vi "UHR-Fleezers Control (host) - 10.3.vi"() -> ()   [LabVIEW 2010]
uses:
  <vilib>/Utility/miscctls.llb/LVPoint32TypeDef.ctl
  <vilib>/Utility/miscctls.llb/LVMinMaxIncTypeDef.ctl
  openfpgaref.8.6.ctl
  <vilib>/userDefined/High Color/nirio_resource_hc.ctl
  <vilib>/Platform/TimedLoop/XDataNode/XDataNode.xnode
  <vilib>/Platform/TimedLoop/XDataNode/timing_clust.ctl
  <vilib>/Platform/TimedLoop/XDataNode/nitl_modes.ctl
  <vilib>/Platform/TimedLoop/XDataNode/wakeup.ctl
  <vilib>/rvi/interface/nirviOpenFPGA/nirviOpenFPGA.xnode
  FPGA Bitfiles/UHR-FleezersInst_FPGATarget_UHR-FleezersCont_0F5B06C4.lvbitx
  UHR-Fleezers Control (fpga) - 10.3.vi
  <vilib>/rvi/ClientSDK/nirviWhatTheDeviceIsDoing.ctl
  <vilib>/rvi/interface/nirviMethod/nirviMethod.xnode
  <vilib>/rvi/interface/nirviReadWriteControl/nirviReadWriteControl.xnode
  <vilib>/rvi/interface/common/niFpgaNodeNameForErrorReporting.ctl
  <vilib>/rvi/errors/niLvFpgaWhatHappensToTopLevelVI.ctl
  <vilib>/express/express analysis/Spectral/XNode/ExpressSpectralMeasurementsBlockNode.xnode
  <vilib>/rvi/interface/nirviCloseFPGA/nirviCloseFPGA.xnode
  <vilib>/Instr/_visa.llb/VISA Configure Serial Port (Instr).vi
  <vilib>/FPGAPlugInAG/PCIe-7852R/niLvFpga_Open_PCIe-7852R.vi
  <vilib>/FPGAPlugInAG/PCIe-7852R/niLvFpga_Reset_PCIe-7852R.vi
  <vilib>/Utility/error.llb/Error Cluster From Error Code.vi
  <vilib>/rvi/errors/niLvFpgaAdjustHostInterfaceError.vi
  <vilib>/express/express analysis/Spectral/Block/exnSpectralBlock spectral measurements PSD poly.vi
  <vilib>/express/express analysis/Spectral/Block/exnSpectralBlock spectral measurements PSD WFM.vi
  <vilib>/Waveform/WDTOps.llb/WDT Append Waveforms DBL.vi
  <vilib>/FPGAPlugInAG/PCIe-7852R/niLvFpga_Close_PCIe-7852R.vi
  <vilib>/Analysis/NI_AALBase.lvlib
  <vilib>/vision/Avi1.llb/AviRefnum.ctl
  <vilib>/Platform/TimedLoop/XDataNode/XDNodeRunTimeDep.lvlib
  <vilib>/vision/NI_Vision_Development_Module.lvlib
  NiFpgaLv.dll
panel:
  in  "Sample Channel Flow":bool
  in  "Pump 3 contents":string="Left: ADig beads" caption="contents"
  in  "Pump 1 contents":string="Right: DNA beads" caption="contents"
  in  "Scripts":T1(tab)=enum."Stepping data"
  in  "Take Stepping Data":bool
  in  "Cap 1 Samp Flow ON":bool=TRUE
  in  "Cap 2 Samp Flow ON":bool=TRUE
  in  "Got DNA bead":bool
  in  "Got ADig bead":bool
  in  "Cap 2 Flow ON":bool=TRUE
  in  "Cap 1 Flow ON":bool=TRUE
  in  "Cap 2 T ON":bool=TRUE
  in  "Move Cap. 2 (ADig Left)":bool
  in  "Move Cap. 1 (DNA Right)":bool
  in  "Cal/Data Acq. Spot":bool
  in  "Dump Beads":bool
  in  "Lower Ch. Cap.":bool
  in  "Cap 1 T ON":bool=TRUE
  in  "Offset 2 Set":dbl=2.0
  in  "Offset 1 Set":dbl
  in  "Cal @ (MHz)":dbl=15.0
  in  "W/ Offset 1":bool=TRUE
  in  "Offset 1 Start (MHz)":dbl=13.0
  in  "W/ Offset 2":bool=TRUE
  in  "Offset 2 Start (MHz)":dbl=16.0
  in  "Move to Delta 2 (MHz)":dbl=13.0
  in  "Attempt Limit":dbl=30.0 caption="Limit"
  out "Attempts":dbl=1.0
  in  "Wait Before Save (s)":u32=1
  in  "Fish for Tether":bool
  in  "Closest Delta (MHz)":dbl=9.5 step=0.25
  in  "Stop F (pN)":dbl=3.0
  in  "Then...":string(combo)="5"
  in  "Move to Delta 1 (MHz)":dbl=13.0
  in  "Tether Alarm?":bool=TRUE
  out "Tether":bool
  in  "TA Cancel Save?":bool=TRUE
  in  "TA Green Off?":bool=TRUE
  in  "Raster Set Upon Tether":u32=1
  in  "Save at end (5, 6)":bool
  in  "N Steps":dbl=20.0
  in  "Step Size (nm)":dbl=0.34
  in  "Save ave factor":dbl=1.0
  in  "Dip Trap Delta 1 (MHz)":dbl=15.0
  in  "Move Trap Before?":bool
  in  "Save Data After?":bool
  in  "Green ON After?":bool
  in  "Dip Trap Delta 2 (MHz)":dbl=15.0
  in  "Move Trap After?":bool
  in  "Duration (s)":dbl=1.0
  in  "Dip for Protein":bool
  in  "APD to Watch":bool
  out "Duration (s)":dbl
  in  "Action":string(combo)="Yank"
  in  "Fl. Triggered...":bool
  in  "Fl. Delta Thresh. (kHz)":dbl=0.6
  out "Waiting":bool
  out "Fl. High":bool
  in  "N pts to average":u16=6
  in  "Yank Delay (s)":dbl=3.5
  in  "Yank to Delta Array (MHz)":dbl[](array[numeric])=[16.3, 15.85, 14.85]
  in  "N Array El":u8=3 min=1 step=1
  in  "Random Choice":bool=TRUE
  in  "Force Yank":bool
  in  "Force Reset":bool
  in  "Y change (mm)":dbl
  in  "Profile":bool
  out "Current Position":cluster{dbl, dbl, dbl}
  out "Sigma/Mean 2":dbl=nan caption="Sigma/Mean" format="%#_2g"
  out "Rate sigma (Hz) 2":dbl caption="Sigma (Hz)" format="%0.2f"
  out "APD 2 Rate (Hz)":dbl format="%#_3p"
  out "Primary Video Display":T2(plugin-control)
  out "Waveform Graph":dbl[](graph) caption="APD Line Scan"
  in  "Inject Pump 3":bool
  in  "Inject Pump 1":bool
  out "Messages":string="4:54 PM\tLost tether (723 s).\r4:42 PM\tFormed tether in 1 attempt(s).\r4:41 PM\tLost tether (470 s).\r4:34 PM\tFormed tether in 7 attempt(s).\r4:32 PM\tLost tether (992 s).\r4:15 PM\tFormed tether in 1 attempt(s).\r4:14 PM\tLost tether (454 s).\r4:06 PM\tFormed tether in 5 attempt(s).\r4:05 PM\tLost tether (206 s).\r4:01 PM\tFormed tether in 3 attempt(s).\r4:00 PM\tLost tether (153 s).\r3:57 PM\tFormed tether in 5 attempt(s).\r3:56 PM\tLost tether (759 s).\r3:43 PM\tFormed tether in 17 attempt(s).\r3:39 PM\tUHR-Fleezers ready.\r"
  in  "APD Ave N":dbl=10.0
  out "Int. Time (s)":dbl=3.0
  in  "Stop All":bool=TRUE
  out "Sigma/Mean":dbl=nan format="%#_2g"
  out "Rate sigma (Hz)":dbl caption="Sigma (Hz)" format="%0.2f"
  in  "Tab Control 6":T3(tab)
  in  "APD 2 Offset":dbl
  in  "APD 1 Offset":dbl
  out "RMS (Ang)":dbl=2.2363215515597568 format="%_2g"
  in  "Bead Sep. Int. Time (s)":dbl=5.0 caption="Int. Time (s)"
  in  "Below (kHz)":dbl=0.5
  in  "Above (kHz)":dbl=2.0
  in  "Adjust Scale\nto Mean":bool
  in  "Rescale on Mean":bool
  in  "Offset (nm)":dbl
  out "Mean":dbl=0.35502251163091847 caption="Mean (pN)" format="%#_3g"
  out "Force":waveform(dbl)[](graph)=[{"t0"=timestamp(4478.100000001255 s since 1904-01-01), "dt"=0.15, "Y"=[0.6544682133105884, 0.6829563430169571], "attributes"=variant("NI_ChannelName"=variant(string "T1 X"))}, {"t0"=timestamp(4478.100000001255 s since 1904-01-01), "dt"=0.15, "Y"=[0.05685503756215739, 0.025810452633971234], "attributes"=variant("NI_ChannelName"=variant(string "T2 X"))}]
  out "APD Chart":waveform(dbl)[](graph)=[{"t0"=timestamp(4478.100000001255 s since 1904-01-01), "dt"=0.15, "Y"=[0.0, 0.0], "attributes"=variant("NI_ChannelName"=variant(string "APD 1"))}, {"t0"=timestamp(4478.100000001255 s since 1904-01-01), "dt"=0.15, "Y"=[0.0, 0.0], "attributes"=variant("NI_ChannelName"=variant(string "APD 2"))}]
  in  "Calibration":u16(ring)=2 items=["None", "Position", "Force"]
  out "T1 X":dbl=0.6687122781637727 caption="T1 X (pN)" format="%0.2f"
  out "T2 X":dbl=-0.04133274509806431 caption="T2 X (pN)" format="%0.2f"
  out "Bead Separation":waveform(dbl)(graph)={"t0"=timestamp(4478.100000001255 s since 1904-01-01), "dt"=0.15, "Y"=[-2.9090620115549504, -2.8815158675481127], "attributes"=variant("NI_ChannelName"=variant(string "T1 X"))}
  in  "Amplitude (nm)":dbl=3.0
  out "Bead Mean (nm)":dbl=-2.9725093766937554 caption="Mean (nm)" format="%0.2f"
  out "Difference":dbl=0.6273795330657084 caption="Difference (pN)" format="%.2g"
  in  "Take Detection Laser\nImage":bool
  out "APD 2":T2(plugin-control) caption="APD 2 (Cy5)"
  in  "Flip Green Filter":bool
  in  "Set X Only":bool
  in  "Set Y Only":bool
  out "APD 1":T2(plugin-control) caption="APD 1 (Cy3)"
  out "Detection Laser Y":T2(plugin-control)
  out "Pointer Y (V)":dbl format="%_3g"
  out "Pointer X (V)":dbl format="%_3g"
  in  "Set Confocal Spot (X-Y)":bool
  out "Detection Laser X":T2(plugin-control)
  out "Saved APD":dbl[][](graph) caption="Most Recent Time Trace"
  out "Trap Delta Graph":dbl[](graph)=[-89.38744840610437, -89.37006347356015, -89.24966097161428, -89.27535644051642, -89.22559285551776, -88.86555051929984, -88.57164165504085, -88.51902465601101, -88.63501771008777, -89.20867383045751, -89.55461281382372, -89.55813284408976, -89.07876691073398, -89.12824891342606, -88.87613266846802, -89.2801470410057, -89.52897456305874, -89.30818962554463, -89.2603892282628, -89.55143394553988, -89.11898533922138, -89.25742201435101, -88.7246017921867, -89.05704019082833, -89.00438612954582, -89.05564776220227, -89.01771654795576, -88.8637677243877, -88.73420125440117, -88.90230035101814, -88.93449064288166, -88.68475787636112, -88.71497640229151, -88.98867971389947, -88.98987818265206, -88.8663554218612, -89.21049798942109, -88.87888603452649, -88.83494841134385, -88.8517410807533, -88.94938680318202, -88.98692447842114, -89.13767155188884, -89.05931890170092, -89.08641661114396, -89.05365179724527, -89.20227840355159, -89.31178251999566, -89.45607605619048, -88.83940363384923, -89.15369570967569, -89.08546468517298, -89.05175431278485, -88.87130156752026, -89.02771493961416, -89.34443740021561, -89.4552359343601, -89.16107171540548, -89.11889587027639, -89.3436162545047, -89.33942660204508, -89.3473584178231, -89.19585027499929, -89.139379143746, -89.2555989459276, -89.20141717607427, -89.21660561984382, -89.46769272591796, -89.07315603501014, -89.03933689450355, -89.0993712485838, -89.35756915821324, -89.35331075709209, -89.22317576092196, -89.508816612592, -89.2518218067191, -89.20936039087964, -89.44092145450193, -89.6477278697556, -89.08293610392039, -89.53347805395603, -89.64410456441405, -89.35761400349834, -89.34886843709035, -89.37851091701371, -89.41649939174766, -89.36071107503787, -89.57311912534034, -89.63101869252588, -89.43405030861993, -89.31069880452256, -89.3430526304503, -89.21823174554396, -89.21501556105062, -88.9111722206407, -89.18733719432157, -89.18722963976052, -89.32292422573383, -89.39588663013811, -89.82453679095343, -89.10638459364176, -89.47188371738739, -89.54185028737668, -89.5729147724991, -89.54460422995446, -89.18025179411762, -89.34220054522804, -89.5575088561865, -89.42069201414144, -89.26950662803745, -89.10557494488836, -89.34610419003715, -89.49955675225459, -89.22456738111956, -89.2027117963072, -89.1349219342003, -89.14160870895898, -89.33136024231399, -89.33342512716312, -89.37714552414755, -89.3803929736005, -89.35573543764183, -89.52038271838603, -89.27965821960461, -89.35600452793587, -89.22650740978278, -89.22614620509182, -89.12635779184048, -89.48788165476256, -89.13068590269111, -89.17357255767598, -89.08072258562063, -88.86940497190369, -88.77122041116284, -88.99968531958817, -89.00921784902013, -88.81448561314173, -88.84031989144572, -89.39146413421481, -88.86339059547717, -89.1673772901552, -89.15159384824292, -89.06085219395777, -89.51260432037202, -89.5536217833934, -88.98677652908017, -89.2701030586531, -89.24195272293136, -89.71292340734871, -89.2910030757885, -89.47786455696955, -89.48954430167501, -89.26584207463125, -89.10233578501436, -89.17707533292848, -89.305147933605, -89.18901651866418, -89.34296303989353, -89.09380910376896, -89.463391307056, -89.57679916102225, -88.71111300258505, -88.94498405110207, -88.49140535622053, -88.7341514685107, -88.89889681017223, -88.59002712151397, -88.76524603655983, -88.87121714891552, -89.1510876045764, -88.91862351911718, -88.82548575374531, -88.80051417887705, -88.54837294030075, -88.87140478869503, -88.89456579635265, -89.0056346348357, -88.55907846911137, -88.66759749781659, -88.44149474414237, -88.6870846816969, -88.6466799778529, -88.63814297254739, -88.78805261976106, -88.96824024662688, -89.1103699249511, -89.3905085878867, -88.9323741748437, -88.75430601059085, -88.82089140957092, -89.4535647245052, -88.85616866717044, -88.79523221810146, -88.9348514263713, -89.16871433406047, -88.67265636299146, -88.56040235473944, -88.91232897311664, -88.8089571372157, -88.91314583351732, -88.88683122051, -88.68204457129616, -88.85998808560862, -89.14884267359204, -89.22322206568205, -88.95108210276138, -88.64718246491319, -89.13249650680967, -88.76829543884, -88.95527962559021, -89.21056707808899, -89.0089527300235, -88.91866866096028, -88.80863987306557, -88.80089852688, -88.78342735706066, -88.56360335694336, -88.67735013119068, -88.59275253806658, -88.69077558769106, -89.13757241655324, -88.73750458538608, -88.78152831683693, -88.99066615201534, -88.82091590097372, -88.82476418112773, -88.85316711473837, -88.66503995216488, -88.79388285985826, -88.9563338555671, -88.71352135994421, -88.83999603213721, -88.74633806352192, -88.60900128977838, -88.53872550741977, -88.18424116231269, -88.3705578352791, -88.62148742046897, -88.54394496460543, -88.36251412656927, -88.4093878967337, -88.50258216055909, -88.35494559212471, -88.34341283426755, -88.37395270939074, -88.4979905289099, -88.46189758015758, -88.26844057461545, -88.2326502387395, -88.55042578244075, -88.63499132099773, -88.51319899426838, -88.73389987228151, -88.26715288988908, -88.21859961845635, -88.58277595542361, -88.59002127369436, -88.55251451009755, -88.37746006671004, -88.41015869076773, -88.51995467108634, -88.20521115956211, -88.2804480699595, -88.43819946605072, -88.33640124221915, -88.6531593764619, -88.34679755650652, -88.52043428631671, -88.95056941775016, -89.15761826470202, -89.0652452180153, -89.29976884961121, -89.28829699493275, -88.2664323951737, -88.30873224535377, -88.44209877116936, -88.24099191432931, -88.22287833843131, -88.29139893670066, -88.46447280750237, -88.3910852296664, -88.29985148131229, -88.30822091752688, -88.28362819582696, -88.48902213455159, -88.54998575425876, -88.60669758609019, -88.49144847059677, -88.16296003837576, -88.51396970073476, -88.33982443813122, -88.22394802157045, -88.29260704896129, -88.41055824500185, -88.33497551461949, -88.67759606488578, -88.58700366093623, -88.35694653040895, -88.47296601718023, -88.33423129919967, -88.47752188464662, -88.35512247733888, -88.3777986712967, -88.729655522916, -88.73598917774595, -88.51630362857102, -88.2074894465274, -88.29181479700983, -88.4672686755314, -88.16849552794635, -88.5951381838874, -88.13062428528687, -88.17216964798284, -88.10524634348789, -88.27800416343854, -88.13335451761374, -88.37825316932381, -88.56140566187452, -88.4425002811831, -88.0656866086508, -88.42547083397028, -88.25095406936146, -88.30824818401392, -87.68332283229768, -88.17932407982077, -88.1532062150512, -88.53375395739056, -88.30311164463794, -88.41589198652929, -88.30407778660808, -88.40367169747444, -88.3437214846239, -88.35594639765567, -88.45652784227724, -88.5842630911653, -88.41297448484298, -88.54859586632723, -88.58103611816637, -88.84792541633075, -88.01907631016554, -87.95324520506506, -87.78481343426844, -87.95560385851115, -87.85804482449285, -88.18551136231898, -88.01656053816524, -88.02895257484454, -87.92828548442509, -87.79710285471337, -88.00738538313797, -87.73682830549747, -88.07275568855894, -87.99433270558389, -87.72770755009651, -87.9267710314997, -87.96904944990774, -87.9253259336599, -88.05705393409421, -88.01203421488725, -87.91328847459181, -87.8071326736109, -88.01735651800155, -88.01900222553235, -87.9545136667229, -88.12450941379944, -87.93910654707737, -87.87354402092201, -87.92735293954016, -88.19340411458231, -88.30401091141142, -87.95775584337821, -87.73163787609764, -88.15344693968393, -87.96650228747762, -88.11064491691332, -87.54860462573924, -88.09354412638375, -87.8519133361432, -87.85881854278162, -88.20509785833131, -87.91760524446005, -87.95035519016639, -88.04278622326103, -88.02524699015602, -88.15194655200104, -88.00407435605808, -88.05793027060378, -87.77335005358424, -88.16544477454528, -87.89450200769897, -88.13982524656109, -87.97826541537938, -88.16268206508684, -87.71879293293877, -87.94985415206207, -87.8064061100325, -87.99934582850895, -88.22615609606846, -87.86093151137626, -87.6700537142207, -88.03078580167295, -87.87513742989012, -87.82347052576961, -87.94732046431275, -88.1156839391357, -88.20232764763225, -88.2994531521694, -88.18386916539099, -88.09031322297545, -88.15313742433287, -87.80239936551692, -87.60250611850887, -87.64533018569459, -87.60991041695632, -87.72676066199486, -87.33559917500989, -87.45284913194946, -87.25817364254561, -87.65430559235227, -87.53602431965585, -87.39786877894335, -87.58615486117924, -87.43227285896955, -87.71344886287676, -87.23377729485536, -87.64014203399677, -87.60239562637292, -87.2919811059202, -87.37115314323583, -87.37275952371664, -87.15051723589367, -87.39185774051927, -87.48653698268699, -87.45749749831653, -87.18067937552632, -87.27483719659506, -87.41864167455336, -87.25027078789361, -86.98471314584748, -87.28270035864435, -87.57027222590403, -87.7665499148163, -87.37999966120944, -87.28971186976376, -87.52306556218589, -87.36410821351811, -87.48529464229739, -87.44136200138482, -87.58907511569913, -87.78643723152783, -87.55681182743275, -87.48385705148843, -87.63330822003329, -87.61184020150489, -87.71616882826622, -87.5282648586323, -87.57071058488614, -87.57236293781206, -87.31757130397664, -87.77813876094464, -87.6257729513794, -87.69068528914049, -87.84520252155934, -87.86085934550638, -87.88195380904611, -87.60311641516779, -87.69122196636401, -87.8020108027814, -87.83361495277228, -87.67067092860452, -87.58389183513452, -87.56129213793758, -87.85975339337645, -87.40220585601887, -87.91728954021838, -87.75864018540607, -87.74689815457056, -87.68245059351156, -88.18451430943892, -87.88738917293477, -87.63757611994254, -87.5708434435605, -87.77278345407868, -87.93142286703629, -87.86352661774805, -87.76673769548492, -88.01908196291075, -87.89074636276199, -87.72684473268411, -87.57289839262214, -87.71597780604532, -87.78577424237625, -87.69032008091057, -87.62589406030267, -87.8174289613667, -87.67707669627433, -87.51845749917389, -87.71466525148008, -87.5606836249847, -87.7139674908129, -87.74094794957122, -87.7005157479694, -87.76640578300322, -87.70527246506592, -87.71611718410986, -87.81476293350636, -87.79251662258699, -87.88265447337088, -87.75795727658604, -87.9823722895671, -88.0836963787135, -87.62714330665065, -88.0089934508544, -87.40707301914264, -88.05177962004032, -87.8229318229869, -87.94390489036448, -87.84493365424993, -87.59509612382958, -87.72856415566281, -87.81497085062107, -87.92128557509571, -87.75918240002704, -87.93548815031771, -87.9012355596515, -87.54139193308774, -87.55828881541663, -87.51056903539299, -87.52039866561812, -87.63682624093673, -87.5432671707731, -87.64742561154168, -87.3288423556632, -87.48046022363206, -87.58910493044621, -87.6911525123038, -87.37349047159623, -87.4448807965905, -87.28808399952601, -87.54929046394128, -87.45969579508173, -87.58502984558035, -87.80226057043029, -88.0303971858355, -87.60810918962494, -87.84113021898624, -87.54927790962793, -87.56484012122169, -87.28054131732654, -87.70220256814717, -87.76341332349702, -87.54370605152829, -87.79205016647634, -88.09313027253401, -88.0620175534996, -87.94063041986826, -87.96896727307845, -87.80256403811197, -87.67239701062852, -87.6399317276719, -87.65889725479741, -87.28729774193249, -87.5214594744474, -87.62016692063344, -87.62735969457016, -87.45027005933, -87.21012664990556, -87.06867512023265, -87.33435958229319, -87.3177444330734, -87.34788825501778, -87.56436416954135, -87.61950903708983, -87.55425148575165, -87.55083323246308, -87.68012788709825, -87.51834206500418, -87.69598428135353, -87.71876397280123, -87.44913472298718, -87.6048484121969, -87.864444966875, -87.5501946692936, -87.45216722120793, -87.58237945926253, -87.78969615154085, -87.67686931387769, -87.5522680359406, -87.44068603371, -87.76799995194563, -87.60672463029596, -87.38968106380253, -87.63066293473824, -88.02940059078153, -87.86955200993, -87.9565636486737, -86.8106204704307, -87.18970625895963, -87.86114644151831, -87.58153303504436, -87.35048262951038, -87.51654038824094, -87.52922696429981, -87.36262242324574, -87.41629136303413, -87.28824237872385, -87.4798012921965, -87.41374424314733, -87.49898141290439, -87.49418606631315, -87.51862153043166, -87.71063407904339, -87.6430033186609, -87.57827338876646, -87.54690816845391, -87.37313105200109, -87.46919199453606, -87.25478433494307, -87.57636908224944, -87.58441520954747, -87.54338977306715, -87.67092323117731, -87.75299003095911, -87.48833905986369, -87.68958700633844, -87.45965031693086, -87.66116717927812, -87.27532000081274, -87.57990013934989, -87.3358908739909, -87.50397985078497, -87.46173599047975, -87.48897346231755, -87.72646057917159, -87.92686417098798, -87.66179360238937, -87.71096805882274, -87.58618277512232, -87.6988941155976, -87.5326287528062, -87.80961641383038, -87.30238479981065, -87.03358687200033, -87.2089031253125, -87.2851268921435, -87.57229679049586, -87.6250778220362, -87.63097627402095, -87.57340931013754, -87.37087860062384, -87.44919654211628, -87.55770928649892, -87.32390714182918, -87.3792060612991, -87.82257062874059, -87.91123683327902, -87.65663152557195, -87.45233009538237, -87.4503607791947, -87.44856346726229, -87.54674508286985, -87.48734914385216, -87.53493633794486, -87.77322141957666, -87.5360093515083, -87.92890453759716, -87.74937580384537, -88.0245676727105, -87.68532561768353, -87.63053250593893, -87.78213147465999, -87.78859059897012, -87.86455124009606, -87.82301747913752, -87.74384895388138, -87.53642726658066, -87.70265895169524, -87.6807943581295, -87.67232336986555, -87.55827287052955, -88.07948443555617, -87.63008108422747, -87.5546049107237, -88.02124763911905, -87.79747135539168, -87.69866730651353, -87.4907995965221, -87.66252496338981, -87.66651266475806, -87.32618843167079, -87.56224440214163, -87.7667193383105, -87.67475148682402, -87.67403549332289, -87.95538747106701, -87.84275776737468, -87.87501919379514, -87.71447099135949, -87.38634807332252, -87.67076191051662, -87.5610535281519, -87.72945280500126, -87.77329172363045, -87.58111844851547, -87.392924048304, -87.99966297359707, -87.66302572401112, -87.70180504315596, -87.7633988137739, -87.49898068274233, -87.60398327290125, -87.55264054889946, -87.7317147994365, -87.44896090874326, -87.73988451581835, -87.6824066023823, -87.7957256934875, -87.61022656628427, -87.63754876347582, -87.5711889574363, -87.81578244682522, -87.51567128404804, -87.5154423142066, -87.52661520916558, -87.90110240253, -87.72240271355116, -87.68284011358159, -87.47969610871385, -87.59549328973137, -87.49486631433797, -87.46292721937864, -87.53242593240981, -87.45177658061101, -87.49650273688985, -87.42222432382316, -87.40924809559812, -87.46155584573685, -87.67740538525773, -87.56795415780982, -87.38569221168117, -87.72497836510254, -87.63212095662197, -87.84874086155294, -87.68423502594806, -87.69248881745025, -87.55053270519312, -87.63792276742947, -87.79361374259113, -87.82594928518766, -88.02381615123241, -87.78573568385676, -87.627134578756, -87.48447531083156, -87.73805939615202, -87.48798012324937, -87.33294279112297, -87.4083676430875, -87.2125741263701, -87.64422154601172, -87.79647571090814, -87.60503235567646, -87.468032119514, -87.5182669364431, -87.69978210057371, -87.50350852296302, -87.05604169095596, -87.54120213385531, -87.52140297291606, -87.40543345419292, -87.5303247718758, -87.53081075788629, -87.29491010008809, -87.55816400580258, -87.41618663405671, -87.40015492786631, -87.66754109572479, -87.64535395323043, -87.7226826283207, -87.76140908067617, -87.55084152605826, -87.67412930855458, -87.66651847157189, -87.59259808382153, -87.76203239123596, -87.82422546599133, -87.83988157302704, -87.63815911780895, -87.49616243720268, -87.33562809133211, -87.4146581786975, -87.57917461085796, -87.58962249843225, -87.530135156205, -87.09582028024963, -87.24486712722238, -87.41117686085059, -87.43803047596957, -87.73298888735778, -87.54712937634724, -87.46411106964821, -87.54784999696707, -87.56584887970729, -87.4903532769867, -87.51231599593729, -87.33147942981621, -87.36305774594335, -87.89964736785245, -87.53883983178878, -87.53308382106005, -87.47942176100906, -87.56968963749078, -87.69694395129795, -87.60185059154233, -87.40409833135215, -87.48565441094152, -87.45295785173542, -87.8598746465701, -87.63829115936099, -87.72329824070167, -87.57755847822077, -87.34233590638961, -87.2456387390855, -87.69022291588266, -87.73497292018078, -87.67861746974165, -87.86636101340743, -87.86785313484236, -87.63076103469672, -87.73204340004872, -87.79896896759101, -87.81165856747944, -87.78886319309825, -87.47167338848682, -87.79033896032894, -87.7394988120906, -87.3593100996421, -87.67569559372204, -87.77973202885244, -87.55832238989285, -87.79523137457565, -87.47172572986554, -87.69117985917633, -87.8026233792443, -87.68335651454673, -87.71072805299252, -87.35688163306679, -87.68247685399328, -88.04111074383601, -87.71006837060239, -87.56964717410253, -87.67187827443692, -87.39882043046879, -87.49501995524523, -87.29313321533394, -87.58729015911976, -87.27415480591418, -87.553455177222, -87.28462813652112, -87.39034628415033, -87.58108941169114, -87.44564719863513, -87.53436292084444, -87.33001410378813, -87.36337024723107, -87.63510719338177, -87.65980368332251, -87.43363496068739, -87.4255269325382, -87.41182525493925, -87.72815339935283, -87.67216110676736, -87.72283448284864, -87.6723969435237, -87.6560403010696, -87.38016535112635, -87.55609880554229, -87.5762178841565, -87.72026364293265, -87.69566289957541, -87.31489376030962, -87.52499386095835, -87.56560915150533, -87.71637669594824, -87.65296554469052, -87.78329628957886, -87.76052147520979, -87.86389250978719, -87.60691705192471, -87.73801394328754, -87.53083942658031, -87.4768796085828, -87.78184542579447, -87.54612819815853, -87.36965481448632, -87.4204871602231, -87.50661200564672, -87.4524351274625, -87.76563007263547, -87.81140346193699, -87.35314925668533, -86.10503470178419, -89.85266012832051, -89.64460892206411, -89.63573878694366, -89.67437474838317, -89.43897047411551, -89.3737613977331, -89.28788917865882, -89.58069848429386, -89.53810567580396, -89.37138670815206, -89.42570077300456, -89.54084483748144, -89.38127981165223, -89.5094888428512, -89.43628497289689, -89.82742727406759, -89.58878997780671, -89.05083051594639, -89.2715449510282, -89.18302882011236, -89.11757972469984, -89.450025337766, -89.4918182082358, -89.48714535759302, -89.45673286538067, -89.3721865723953, -89.22628822081519, -89.54189155991992, -89.3527578161816, -89.55295636678755, -89.61525268024653, -89.60177253387754, -89.35091333052947, -89.65096893870835, -89.43826482992947, -89.26405785507977, -89.13333984803354, -89.27090710005496, -89.61146885238918, -89.38160521758422, -89.41398091645064, -89.56444238217698, -89.55467011390908, -89.49128237350648, -89.50437810521063, -89.49811847441696, -89.58142008085757, -89.70565907063485, -89.79032016312806, -89.49368126396514, -89.43538457890372, -89.22236432143751, -89.30147719799409, -89.6871672866815, -89.39666762420819, -89.53287835086593, -89.53103400899184, -89.30264681130458, -89.20241016917116, -89.20185024762415, -89.14667769335148, -89.4091163236507, -89.5303897169196, -89.37364072083844, -89.36478136588747, -89.52127318590307, -89.47972650316281, -89.5730482533163, -89.62064623540789, -89.5836723763713, -89.51543500545677, -89.38239305279464, -89.62184644095112, -89.7728958272249, -89.683935508047, -89.67854975684114, -89.50641274850042, -89.66409060311157, -89.22826919030574, -89.5351698052126, -89.52386617594226, -89.5762566923911, -89.12011896829341, -89.39440120296695, -89.31526150363645, -89.40699770807561, -89.27641788881832, -88.9980934526029, -89.22189882622396, -89.18320922801408, -89.07312242319608, -88.83297400882918, -89.2234100301694, -88.85288595229059, -89.2377991335614, -89.35741830027712, -89.26107817432187, -89.43580762503471, -89.41514590200433, -89.45677685231738, -89.34136783820585, -89.21998788359926, -88.86601818955353, -89.36404024707687, -89.18530760698397, -89.43678951078016, -89.18406807997061, -89.37969189195263, -89.62263416697985, -89.37304214824837, -89.3440877767074, -89.3598322726397, -89.34954279527221, -89.19348306086874, -89.2146973031071, -89.43625648517998, -89.34417299103697, -89.52160411222111, -89.53337708387906, -89.342069859851, -89.5743618155725, -89.30272336229824, -89.15741114850327, -89.21817485093237, -89.30503477455262, -89.36081784103939, -89.52459993172579, -89.6111165131166, -89.2619524554189, -89.35664568024671, -89.22996326941124, -89.42804922425438, -89.42197549285336, -89.62869122920705, -89.38083285342586, -89.54868019256227, -89.31926914035074, -89.55393076075502, -89.39585117735736, -89.56232500771125, -89.58429220453907, -89.2853335425489, -88.9554979363846, -89.82366236227894, -90.03241697822503, -89.87535834289318, -89.68803825964758, -89.90985739705187, -89.65052212097332, -89.63592492369258, -89.68901377113175, -89.61580926284557, -89.47648673035042, -89.5763572557888, -89.62979756653974, -89.48581314130413, -89.60156409856245, -89.521773057561, -89.2283702112482, -89.36270907008742, -89.3762029830632, -89.37264199967436, -89.47817702167433, -88.96620231000924, -89.54818090594742, -89.80996257603499, -89.63617690920825, -89.27694912725786, -89.17404501094248, -89.36048391493902, -88.88941872416451, -88.84313652275561, -89.25869975047635, -89.51915145305644, -89.3148346155159, -89.23949602638928, -89.27060642492778, -88.82059631185331, -89.22377299622616, -89.40471068902889, -89.67545363713047, -89.7105622164905, -89.59379751329226, -89.43763803920422, -89.73367902969775, -89.25258989064338, -88.92196116042703, -89.49284759320145, -89.43652161750485, -89.14923694928899, -89.31570366092012, -89.14198709968517, -89.22103878715308, -89.31243636768616, -89.35968282595243, -89.45840321040957, -88.9639394112719, -89.41425315620818, -89.36940537708537, -89.43031076815686, -89.20706343917448, -89.43495800271168, -89.29789897809772, -89.17597071053217, -89.2602152121373, -89.55991216232033, -89.13369209792404, -89.26909295138859, -89.3238551922488, -89.48669087227324, -89.423659006272, -89.50933552398729, -89.60114730778753, -89.36920727072032, -89.20780895747096, -89.67447177677113, -89.88591928368581, -89.34584482112372, -89.44820280802116, -89.49125823457338, -89.6568084287604, -89.43129708145736, -89.19178935178499, -89.28690969251289, -88.84810710672292, -89.40764696202572, -89.98838207910475, -89.46179401598928, -89.96003721353357, -90.29385321683213, -89.60860309937391, -89.06511935921438, -89.03125538678515, -89.51945033113051, -88.9977216866873, -89.23373707873185, -89.21931962136915, -89.87772162313416, -88.81461035446387, -89.41037526458646, -89.21597949792773, -89.12932586845321, -88.89371870329344, -89.33259816499356, -89.40470973446673, -89.3877910698847, -89.29257692524722, -89.76283867032404, -89.10096113503705, -89.0024552709693, -89.3505470549878, -89.37600264393359, -89.26597700316711, -89.5802441405524, -89.57893446891464, -88.91904199379911, -89.3815923013336, -89.18055657100285, -88.96373412987602, -89.15474436507003, -89.05102563118294, -88.91995887489625, -89.07392479076549, -89.34741814351625, -89.87526391116663, -89.19926148148149, -89.119620884163, -89.0393605559567, -88.77208870822894, -89.32195301903197, -89.09069786094281, -89.19673976535732, -89.14714102710515, -89.10779711665595, -89.08023600035908, -89.04761082212389, -89.00208857126661, -88.96839649386507, -88.76778670987548, -89.17048722940753, -89.30230976822241, -89.29160258844252, -89.3333423944874, -89.21683284951314, -89.31454210337398, -89.05934971458657, -89.23120006336663, -88.88610370286466, -88.97987228055663, -89.55143616735391, -89.45064218424297, -89.0965360803919, -89.14366272878738, -89.31218063333657, -89.0432226236395, -89.307677489395, -89.34063352548658, -89.32168023132036, -89.3126281281213, -89.20696593023561, -89.05718230378571, -89.16465103462701, -89.11847781964123, -89.24427371080426, -89.23214449007804, -89.27216161870632, -89.46769195656496, -89.45641376742469, -89.44714253031034, -89.04140792595314, -89.24701195071574, -89.39451905841605, -89.08543130907711, -89.45861193371825, -89.89974996696542, -89.43123387431251, -89.08641401326244, -89.13619110631862, -89.1826801708081, -89.17246493676171, -89.15652161423958, -88.78487650718846, -89.11971463463695, -88.76150695192209, -89.22036295485265, -89.20267147034549, -89.11729408223869, -89.4393059908418, -89.14636436459836, -89.15795395207269, -89.4275262122909, -89.22238485841942, -89.21940749412003, -89.08009114913443, -89.48920642046721, -89.15156442516772, -89.45698509789325, -88.87338314085522, -89.11045757349817, -89.46914647939062, -89.39797361779893, -89.420351098198, -89.38772867407957, -89.53347062365026, -89.25834313541426, -89.41957494353836, -89.29725722999143, -89.32381954159032, -89.39665434288693, -89.27290066010944, -89.49545804363956, -89.27060062024876, -89.3447405329835, -89.08272641196109, -89.305114113685, -89.42518021075358, -89.2482325160118, -89.38755628933976, -89.42168348053734, -89.04454862092464, -89.14915329392596, -89.37450589674879, -89.04039420204515, -89.1981375340063, -89.17596255924028, -89.13528304594989, -89.00356265969344, -89.261399469586, -88.96269949077983, -89.14333106859672, -89.41455145051421, -89.04943284927722, -88.86088894489063, -89.17453593650691, -88.66918119841439, -89.294146960962, -89.00819033468315, -89.04068043481627, -89.17620516400488, -89.09515362657663, -88.95981966328938, -89.15098552560895, -88.86236589470138, -89.21890741278276, -88.98251136025263, -89.03656163327432, -89.06019956154205, -89.23130134405736, -88.85390859847459, -89.22274938143335, -89.31166831425534, -89.76364552125162, -89.69880521261672, -89.34933991804397, -89.40903838807759, -89.11958827058041, -89.34058831435459, -89.64853755096333, -89.15690431343052, -89.45072666387912, -89.13948595908302, -89.40378733596806, -89.4634451436483, -88.0871954402557, -90.2523886297195, -90.32635437152004, -90.24503616401293, -90.17296891811858, -89.96316337641721, -90.19549823074706, -90.23014161336732, -90.13269117603848, -90.13546395158026, -90.24674659520822, -90.40157823810915, -89.73909437391183, -90.096832647288, -90.07515881472611, -90.41954622389525, -90.3825268323373, -90.18163811914361, -90.32412477840575, -90.19229216788813, -90.44522597500249, -90.13766390475877, -89.66968325889837, -89.9126565384995, -90.35605823166685, -90.28443307623621, -90.2234051820104, -90.21097840754392, -90.1434932206816, -90.24664411952034, -90.16297084625032, -89.99669745613257, -90.21337271531756, -90.021247708263, -90.06112766083584, -90.15294351289444, -90.19356620613507, -90.51319106617697, -90.09652105317282, -90.16690415325345, -90.45503996596538, -90.55116792842264, -90.07640911035573, -90.36256889908509, -90.20735243748508, -90.5326486662778, -90.41875749798626, -89.96515492584263, -89.8797442385357, -89.99429197617584, -90.21637803668041, -90.23608863956005, -90.30275101535133, -90.41942234871539, -90.33711424926108, -90.42214648701524, -90.27257976521608, -90.05960656456891, -90.03794536093727, -90.08741347741497, -90.43472618317658, -90.2522644360195, -90.29086269882997, -90.40629287671857, -90.61792619604786, -90.36613512437535, -90.29050508079987, -90.48790384558785, -90.12556116500082, -90.40000509329306, -90.51190694229909, -90.48024005146416, -90.63891561252724, -90.64839317421082, -90.1166652138771, -90.07533432694785, -90.34473101826771, -90.43451148283822, -90.61504799434994, -90.35172125444156, -90.5824314759526, -90.42203000224241, -90.45334459367774, -90.50472974606436, -90.64884364476089, -90.30968289889046, -90.45213831077214, -90.39147347172283, -90.17120557360909, -90.47525243001763, -90.396195657183, -90.31707930262343, -90.48713957741559, -90.42975001686625, -90.29789082657939, -90.46790304802579, -90.0947530517084, -90.328084029011, -90.30997424183043, -90.37316674979998, -90.29985642166363, -90.45006812043209, -90.17167534801723, -90.25468560102487, -90.15474421553142, -89.83393535067671, -90.20056478170406, -90.00296367297801, -90.21273519120342, -90.03490472002353, -89.94516964918006, -90.11067497816705, -90.18166776257632, -89.98882698225557, -89.85974377965816, -90.26505571518203, -90.15363713435593, -89.93316277964567, -89.95255251704741, -90.09698121390325, -90.04473329210172, -90.20534251503767, -90.458225224308, -90.2193790684706, -90.4599285306242, -90.5129940662291, -90.42282464467658, -90.37899575214976, -90.51315578513703, -90.50498529009057, -90.49201239331842, -90.50509139004552, -90.65465381069006, -90.24135716282727, -90.49818058178988, -90.54508650659335, -90.590507880303, -90.22481588702846, -90.44954328100238, -90.42767895442282, -90.40665355719054, -90.46603422132092, -90.22992008635563, -90.40089196820325, -90.2634868147749, -90.10206808676487, -90.536708726445, -90.1142016245376, -90.14149772635739, -90.14744631109205, -89.96547180840015, -90.21348545778108, -90.19073297991473, -90.37810903808769, -90.36879841716365, -90.42386666329647, -90.3715419481675, -90.29534431533034, -90.4028894344913, -90.15910175646306, -90.37091186837088, -90.1514934185192, -90.08503985404151, -90.29758609982272, -90.24521262721103, -90.22694052004285, -90.34910590301128, -90.31444089221904, -90.35215687320854, -90.26487760335966, -90.26219431605509, -89.97109692967945, -90.33087070872675, -90.45526539699613, -90.46167631785531, -90.44946334620084, -90.26650949052697, -90.38637346294726, -90.30254359116161, -89.97816869969462, -90.12232129716138, -91.63843000396554, -89.7362298577711, -89.54498333392092, -89.49938002867206, -89.49058379559563, -89.55044220270838, -89.60560601688277, -90.17027697268526, -89.6463463438765, -89.53794199525763, -89.10021704348154, -89.5457703413785, -89.25321894536543, -89.33345773463982, -89.58058389614905, -89.5168680518304, -89.47368234056128, -89.4058238856133, -89.15141597620514, -89.19282754602571, -89.58609886577267, -89.37019238993713, -89.37365136237787, -89.64303187671761, -89.2393858200982, -88.80127698898539, -89.11581946876925, -89.80767872863254, -88.93708737205955, -88.90962554991867, -88.88195933948012, -89.25706660886158, -89.02345428583934, -89.3022672789113, -89.2838649764038, -89.14654756383041, -88.86384783388766, -88.9175525867171, -89.21412651700874, -89.04860439238527, -89.25613750447775, -88.96517619327935, -89.12360954681394, -89.11224916640745, -89.16770424614049, -89.06094806010964, -89.0191470090751, -89.45687258453175, -89.60591860772492, -89.29585239378879, -89.83889261634286, -89.41013138045021, -89.63967513661015, -89.25797313024034, -89.6814018591188, -89.68821168672036, -89.58541567807737, -89.54188235417723, -89.61661971119183, -89.40723078839817, -89.34843089690773, -89.60515585313834, -89.56246156265125, -89.59370346754119, -89.66038143523066, -89.62559461914364, -89.42478326266355, -89.73029454506324, -89.43000935590837, -89.428288891753, -89.37564130633967, -89.02189968500151, -89.10788041065231, -89.32596209412588, -89.39404483901504, -89.4129768306943, -89.22209321815708, -89.10303797163806, -89.24924057430192, -89.49693081718887, -89.70833547833459, -89.6786839552272, -89.64591606711676, -89.51344631340291, -89.41101181324719, -88.44650019934619, -90.17731549807735, -90.27908072664212, -90.30349753540256, -90.42640638338176, -90.5461620039406, -90.40250304826327, -90.55184676162722, -90.22330217548966, -90.34604266504405, -90.34685720527591, -90.43543106648633, -90.32093998642343, -90.74190071075202, -90.36816598571811, -90.20018695449596, -89.69118008843904, -90.5408534144869, -90.44853203217406, -90.19896449655212, -90.26215618254675, -90.39783468271995, -90.19854594234243, -90.26812455801539, -90.4749038130671, -90.38385254518266, -90.38905614539564, -90.34356884533197, -90.06500891937931, -90.45591618755515, -90.18150542797281, -90.19969514913056, -90.37320685771269, -90.61570682788782, -90.34813631956763, -90.13750975570412, -90.07569812371833, -90.37642677753739, -90.33435317419614, -90.22555657098471, -90.23895375028121, -90.270246205725, -90.37600302883945, -90.2835538905631, -90.28385266083197, -89.78164047619508, -90.196635103456, -90.4809556207527, -90.01232719313069, -90.06390676586018, -90.22571765197469, -90.01167064927066, -90.29315367326132, -90.58357366716768, -90.26604080937142, -90.38515554970854, -90.1664830928737, -90.25566610607, -90.29182101093004, -90.33159656914417, -90.29740664846878, -90.12152543912441, -90.22505748118813, -90.07255937894185, -90.32626829459986, -90.29779540771625, -90.04335682238323, -90.14280906535224, -90.55964225477469, -90.30453958962217, -90.19593466265141, -89.77794966586396, -90.22246406101418, -90.49007992662617, -90.26741236776786, -89.94141182542884, -90.23288838691548, -90.07689253262124, -90.01473799333098, -89.96463099083859, -90.07745323671415, -89.94899441375048, -89.95495681210551, -90.00328638642554, -89.86870577366334, -90.08219568718776, -91.38615529550509, -89.0821447095635, -89.16820375058256, -89.10993184807809, -89.35779724956876, -89.36303709784403, -89.49757924729965, -89.44022066961067, -89.72624177725754, -89.75530879533176, -89.30836834709211, -89.7946009825269, -89.55671449854206, -89.61780451376646, -89.79357732437859, -89.44162363081644, -89.33239502158372, -89.478663009932, -89.66432476618351, -89.4937459042744, -89.41688638394041, -89.44460080624765, -89.43006349407366, -89.53283286899145, -89.48506102868743, -89.40024490411534, -89.32159922616273, -89.49189035607932, -89.0906531149945, -89.57154035461157, -89.3279294963929, -89.5262028900506, -89.4618575942215, -89.04150927193281, -89.23254167591475, -89.32036225135491, -89.52639856617733, -89.6790289190201, -89.8305547288756, -89.23930386276109, -89.5796936157711, -89.32856869184184, -89.48158078475134, -89.72828762784434, -89.32988515382098, -89.82246553111887, -89.1985184370172, -89.53893988629702, -89.54004424539605, -89.31296804318146, -89.40664149900778, -89.4095605730308, -88.90452677109064, -89.27638428969453, -89.4867258866616, -89.30965894808136, -89.05026439296921, -89.20221731059893, -89.15241321656985, -89.03046768602977, -88.97775540843435, -89.35393638033742, -88.87746997687707, -89.01446489393777, -89.42998809448717, -89.41951629723886, -89.29657619825127, -89.66517853351598, -89.26719513501837, -89.19856737181169, -89.31331613858958, -89.20024330138921, -89.68675314326693, -89.18691067885689, -89.44827735606182, -89.56832116008042, -89.3991673752302, -89.35338237886637, -89.19281493368959, -89.5844563456998, -89.59068903809967, -89.58125550151313, -89.55030349938028, -89.48631315915387, -89.49298165244711, -89.19463050450781, -89.41437069631509, -89.12268571079467, -89.18900910332924, -89.3859894958023, -89.25519191016045, -89.66257524290295, -89.33650806620477, -89.20722749651145, -89.38932496965388, -89.29148478789386, -89.39818187499321, -89.15663754761036, -89.5072792261119, -89.32672769334965, -89.57350830973445, -89.05634034293683, -89.00490134040983, -89.01083406418745, -89.37676924966965, -89.21254475296408, -89.03124620071928, -89.39281240345495, -89.33884438506695, -89.33682455468552, -89.49510453196741, -89.2372114044394, -89.55110664840826, -89.46857253003795, -89.05525600766862, -89.51341705464556, -89.49189351125247, -88.69254044548302, -88.8764894755446, -89.17120213281257, -89.22492294329365, -89.63664086781168, -89.74122661974911, -89.42327979427549, -89.55211561515353, -89.33928655995086, -89.30731392907573, -89.42224560331604, -89.21698045572563, -89.30015620250015, -72.02170105722757, 0.14802746146348256, 0.18182087058933108, 0.23145938781077158, 0.3745260603907764, 0.14339761464982548, 0.13744307201019235, 0.1999682238582624, 0.0488607450323251, 0.18909217445305565, 0.15803496802367173, 0.14030285755402744, -0.029758937979426924, -0.07388335400978263, 0.05173577743792419, 0.1120128372807348, -0.18369537610293946, -0.11094340057605118, -0.20700246867226446, 0.10559275090425473, -0.04850788802633353, -0.13341306859012336, -0.175179384438497, -0.147304334629956, -0.046157193510941066, -2.110428849563225, -2.827260759231172, -2.7882000038039294, -3.065306614418958, -2.6738823113174797, -2.840374309742303, -2.8750738677830467, -3.1398929972536034, -3.2420787696181153, -2.909460090063946, -3.322654750798421, -2.9504354301491165, -2.892884216735465, -2.6600659669938373, -2.962705147898145, -2.8667664458259563, -2.9913143616991413, -3.0237422733393706, -3.1941671849037543, -3.100885335284091, -2.648488912011631, -3.1201611300592274, -2.8671399365956125, -2.9393444108016835, -2.889238638161287, -3.067559137434417, -2.907857804168715, -2.715504853234837, -2.943189444947173, -2.749942778041302, -2.765556336531846, -2.8495372144488034, -3.2467998174444275, -3.0843775217642735, -2.7246418838225157, -2.915095163918644, -3.28651986346745, -2.868575252095781, -3.2263560407303267, -2.665341243673598, -2.9235009817725723, -2.7262262496104523, -2.956706675877592, -3.0687540749024307, -2.7511714031298604, -2.6762217304609814, -2.597560824458633, -3.1314839397787306, -2.939241757727324, -3.3114231119313624, -3.083958003204651, -3.018880629301152, -2.6562071342673255] caption="Most Recent Time Trace"
  out "Save APD Deriv":dbl[][](graph) caption="Most Recent Time Trace"
  out "Delta Fl. 1":dbl
  out "Delta Fl. 2":dbl
  out "All Signals":waveform(dbl)[](graph)=[{"t0"=timestamp(4478.100000001255 s since 1904-01-01), "dt"=0.15, "Y"=[0.0, 0.0], "attributes"=variant("NI_ChannelName"=variant(string "APD 1"))}, {"t0"=timestamp(4478.100000001255 s since 1904-01-01), "dt"=0.15, "Y"=[0.0, 0.0], "attributes"=variant("NI_ChannelName"=variant(string "APD 2"))}, {"t0"=timestamp(4478.100000001255 s since 1904-01-01), "dt"=0.15, "Y"=[0.03832069939271974, 0.03825193921460892], "attributes"=variant("NI_ChannelName"=variant(string "T1 Y"))}, {"t0"=timestamp(4478.100000001255 s since 1904-01-01), "dt"=0.15, "Y"=[-0.04115430382333141, -0.04098539428791512], "attributes"=variant("NI_ChannelName"=variant(string "T1 X"))}, {"t0"=timestamp(4478.100000001255 s since 1904-01-01), "dt"=0.15, "Y"=[8.223135319071018, 8.222352671895505], "attributes"=variant("NI_ChannelName"=variant(string "T1 Sum"))}, {"t0"=timestamp(4478.100000001255 s since 1904-01-01), "dt"=0.15, "Y"=[0.049969565217666184, 0.05022434551426698], "attributes"=variant("NI_ChannelName"=variant(string "T2 Y"))}, {"t0"=timestamp(4478.100000001255 s since 1904-01-01), "dt"=0.15, "Y"=[-0.04609831905596902, -0.04591761419661594], "attributes"=variant("NI_ChannelName"=variant(string "T2 X"))}, {"t0"=timestamp(4478.100000001255 s since 1904-01-01), "dt"=0.15, "Y"=[8.16038734092227, 8.159965300454726], "attributes"=variant("NI_ChannelName"=variant(string "T2 Sum"))}, {"t0"=timestamp(4478.100000001255 s since 1904-01-01), "dt"=0.15, "Y"=[0.008344782840181541, 0.008352712723844287], "attributes"=variant("NI_ChannelName"=variant(string "T1 FB X"))}, {"t0"=timestamp(4478.100000001255 s since 1904-01-01), "dt"=0.15, "Y"=[8.999798211615344, 8.999808099612414], "attributes"=variant("NI_ChannelName"=variant(string "T1 FB Sum"))}, {"t0"=timestamp(4478.100000001255 s since 1904-01-01), "dt"=0.15, "Y"=[0.01562539899484444, 0.015629296930858246], "attributes"=variant("NI_ChannelName"=variant(string "T2 FB X"))}, {"t0"=timestamp(4478.100000001255 s since 1904-01-01), "dt"=0.15, "Y"=[8.999790185247353, 8.999797753837703], "attributes"=variant("NI_ChannelName"=variant(string "T2 FB Sum"))}, {"t0"=timestamp(4478.100000001255 s since 1904-01-01), "dt"=0.15, "Y"=[-4.908334489551589, -4.898547275139339], "attributes"=variant("NI_ChannelName"=variant(string "PSD Y"))}, {"t0"=timestamp(4478.100000001255 s since 1904-01-01), "dt"=0.15, "Y"=[-0.42967373813057286, -0.42906247102062434], "attributes"=variant("NI_ChannelName"=variant(string "PSD X"))}, {"t0"=timestamp(4478.100000001255 s since 1904-01-01), "dt"=0.15, "Y"=[-0.019742362743003634, -0.019780571916867582], "attributes"=variant("NI_ChannelName"=variant(string "PSD Y Sum"))}]
  in  "Signals to Plot":i32(listbox)
  out "Trap Disp. Freq. (Hz)":dbl=6.666666666666667 caption="Freq. (Hz)" format="%#_6p"
  out "Display Period (s)":dbl=0.15 caption="Period (s)" format="%#_6p"
  in  "Trap Disp. Downsample":dbl=10000.0 caption="Downsample" max=20000.0
  in  "APD Disp. Scale":dbl=0.1 caption="Scale (Divide,\nfor above plot only)"
  in  "APD Disp. Downsample":dbl=15.0 caption="Integrate" min=1.0 max=30.0 step=1.0
  out "APD Display Freq. (Hz)":dbl=6.666666666666667 caption="Freq. (Hz)"
  out "APD Display Period (s)":dbl=0.15 caption="Period (s)"
  out "FFT 1":cluster{"f0":dbl, "df":dbl, "magnitude":dbl[]}[](graph)=[{"f0"=0.0, "df"=3.3333333333333335, "magnitude"=array[10000 elements]}, {"f0"=0.0, "df"=3.3333333333333335, "magnitude"=array[10000 elements]}]
  out "FFT 2":cluster{"f0":dbl, "df":dbl, "magnitude":dbl[]}[](graph)=[{"f0"=0.0, "df"=3.3333333333333335, "magnitude"=array[10000 elements]}, {"f0"=0.0, "df"=3.3333333333333335, "magnitude"=array[10000 elements]}]
  in  "FFT 1 Choice 1":u16(ring) items=["T1 Y", "T1 X", "T1 Sum", "T2 Y", "T2 X", "T2 Sum", "T1 FB X", "T1 FB Sum", "T2 FB X", "T2 FB Sum", "PSD Y", "PSD X", "PSD Y Sum", "none"]
  in  "FFT 2 Choice 1":u16(ring)=3 items=["T1 Y", "T1 X", "T1 Sum", "T2 Y", "T2 X", "T2 Sum", "T1 FB X", "T1 FB Sum", "T2 FB X", "T2 FB Sum", "PSD Y", "PSD X", "PSD Y Sum", "none"]
  in  "FFT 1 Choice 2":u16(ring)=1 items=["T1 Y", "T1 X", "T1 Sum", "T2 Y", "T2 X", "T2 Sum", "T1 FB X", "T1 FB Sum", "T2 FB X", "T2 FB Sum", "PSD Y", "PSD X", "PSD Y Sum", "none"]
  in  "FFT 2 Choice 2":u16(ring)=4 items=["T1 Y", "T1 X", "T1 Sum", "T2 Y", "T2 X", "T2 Sum", "T1 FB X", "T1 FB Sum", "T2 FB X", "T2 FB Sum", "PSD Y", "PSD X", "PSD Y Sum", "none"]
  in  "Compute FFT":bool=TRUE
  in  "Reset FFT":bool
  in  "# Spectra to Ave.":dbl=25.0
  out "Ave. Time (s)":dbl=7.5
  out "1 Channel":waveform(dbl)(graph)={"t0"=timestamp(0 s since 1904-01-01), "dt"=1.4999999999999999e-05, "Y"=array[20000 elements], "attributes"=variant("NI_ChannelName"=variant(string "T1 Y"))}
  out "Slow mean":dbl=0.04741485510254009 format="%0.2f"
  in  "Slow mean N ave.":dbl=1.0 min=1.0 step=1.0
  out "Mean Intensity":dbl=0.04741485510254009
  out "Sigma":dbl=0.006116447585273888
  out "Sigma/Mean":dbl=0.12899855060289364
  in  "Subtract mean":bool
  in  "High Res. Display":u16(ring) items=["T1 Y", "T1 X", "T1 Sum", "T2 Y", "T2 X", "T2 Sum", "T1 FB X", "T1 FB Sum", "T2 FB X", "T2 FB Sum", "PSD Y", "PSD X", "PSD Y Sum"]
  out "APD 1 Rate (Hz)":dbl format="%#_3p"
  in  "Tab Control":T4(tab)
  out "Stage Moving":bool
  in  "Read Cal":bool
  in  "Confocal Linescan":bool
  in  "Speed (nm/s)":dbl=100.0
  in  "Furthest Withdraw (MHz)":dbl=15.0
  in  "Confocal Image":bool
  in  "Round T1 X":bool caption="Round"
  in  "T1 offset_x (mV)":dbl=-45.0347243000155 format="%#_2g"
  in  "T1 kappa_x (pN/nm)":dbl=0.2471971927099238 min=0.0 step=0.001 format="%#_2g"
  out "Time (s)":dbl=279.9
  out "Total Time (s)":dbl=60.0
  in  "Start Saving":bool
  in  "Cal sets to save":u32=50 min=1 step=1
  in  "Comment (data description)":string="testing confocal setup"
  out "Calibrating Trap...":bool
  in  "Trap 2 (ON/OFF)":bool=TRUE
  in  "Trap 1 (ON/OFF)":bool=TRUE
  in  "Save Calibration":bool
  in  "N sets to save":u32=200 caption="N Sets"
  in  "Save N Sets":bool
  out "Save file name":path=path "E:/Data/101028/101028_052.dat"
  in  "Save ave N":dbl=500.0 caption="Averaging Factor"
  out "Saving...":bool
  in  "Stop Saving":bool
  out "Progress":u16(slide) scale=0.0..100.0
  out "Manipulating Trap":bool
  out "Buffer Status":dbl(slide) scale=0.0..1.0
  out "Overflow (data lost)":bool
  in  "Reset":bool
  out "Data Rate (Hz)":dbl=66666.66666666667 caption="Trap Data Rate (Hz)" format="%#_3p"
  out "Data Period (s)":dbl=1.4999999999999999e-05 caption="Trap Data Period (s)" format="%#_6p"
  out "Save Data Rate (Hz)":dbl=133.33333333333334 caption="Rate (Hz)" format="%#_6p"
  out "Save Data Period (s)":dbl=0.0075 caption="Period (s)" format="%#_6p"
  in  "T1 alpha_x (nm/V)":dbl=682.2856484824291 step=10.0 format="%#_3g"
  in  "T2 alpha_x (nm/V)":dbl=790.1873608955543 step=10.0 format="%#_3g"
  in  "T2 kappa_x (pN/nm)":dbl=0.2174132196053945 min=0.0 step=0.001 format="%#_2g"
  in  "T2 offset_x (mV)":dbl=-45.767376265464655 format="%#_2g"
  in  "BD 1 Frequency 2 (MHz)":dbl=85.0 caption="T2 X (MHz)" min=60.0 max=90.0 step=1.0 format="%#_6p"
  in  "Green Laser ON/Interlacing":bool
  in  "Round T2 X":bool caption="Round"
  in  "AO1":dbl(slide)=6.408063513378007 caption="Confocal Y (V)" min=0.0 max=10.0 step=0.01 scale=0.0..10.0 scale format="%_1f"
  in  "AO2":dbl(slide)=2.4332770775475328 caption="Confocal X (V)" min=0.0 max=10.0 step=0.01 scale=0.0..10.0 scale format="%_1f"
  in  "Trap Raster Scan":bool
  out "Raster Scanning...":bool
  in  "Trap Delta (MHz)":dbl=15.0
  in  "Setpoints (V)":cluster{"Set 1":dbl, "Set 2":dbl}={"Set 1"=9.0, "Set 2"=9.0}
  in  "Index":dbl=52.0 caption="Save File Index" min=1.0 step=1.0
  in  "BD 1 Frequency 1 (MHz)":dbl=70.0 caption="T1 X (MHz)" min=60.0 max=90.0 step=1.0 format="%#_6p"
  in  "Position Label 5":string="upper flow spot (UvrD)" caption="5"
  in  "Move to Position":bool
  in  "Position":dbl=1.0 min=1.0 max=10.0 step=1.0
  in  "Set Position":bool
  in  "Saved Stage Positions":dbl[][](array[numeric])=[[1.0, 2.24438, -0.22402, 0.00732], [2.0, 0.0, 0.0, 0.0], [3.0, 2.75063, -0.30498, 0.00732], [4.0, 2.75063, 0.39507, 0.00732], [5.0, 2.75063, -2.32612, 0.00732], [6.0, 0.0, 0.0, 0.0], [7.0, 0.0, 0.0, 0.0], [8.0, 0.0, 0.0, 0.0], [9.0, 0.0, 0.0, 0.0], [10.0, 0.0, 0.0, 0.0]]
  in  "Move to Position 5":bool
  in  "z nudge increment (um)":dbl=0.5
  in  "+z":bool
  in  "Position 1 Label":string="Right capillary (DNA beads)" caption="1"
  in  "Set Position 1":bool
  in  "Set Position 2":bool
  in  "Set Position 3":bool
  in  "Set Position 4":bool
  in  "Move to Position 3":bool
  in  "Move to Position 4":bool
  in  "Move to Position 2":bool
  in  "Move to Position 1":bool
  in  "Position 2 Label":string="Left capillary (ADig beads)" caption="2"
  in  "Position 3 Label":string="lower flow spot (ATP)" caption="3"
  in  "Position 4 Label":string="Dump beads" caption="4"
  in  "-z":bool
  in  "Set Position 5":bool
  out "Stage Control Serial Error":errorcluster={"status"=FALSE, "code"=1073676293, "source"="VISA Read in Set Stage Position.vi->UHR-Fleezers Control (host) - 10.2.vi"}
  out "Pump 3 cont disp":string="Left: ADig beads"
  out "Pump 1 cont disp":string="Right: DNA beads "
  in  "Ch 1 Inject Rate (ul/h)":dbl=50.0
  in  "Pump write delay (ms)":dbl=300.0
  in  "All Pump Parameters":T5={"Pump 1"={"Diameter (mm)"=4.61, "Units"=4.0, "Volume"=100.0, "Rate"=50.0}, "Pump 2"={"Diameter (mm)"=4.61, "Units"=3.0, "Volume"=0.0, "Rate"=0.0}, "Pump 3"={"Diameter (mm)"=4.61, "Units"=4.0, "Volume"=100.0, "Rate"=250.0}}